vi "UHR-Fleezers Control (host) - 12.7c.vi"() -> ()   [LabVIEW 2012] (continued)
                  n359 = local read "Stop All"() -> (w575:bool)
                  n360 = Or(x=w577, y=w572) -> (x .or. y?=w574:bool)
                  n361 = Not(x=w574) -> (.not. x?=w576:bool)
                  n362 = Compound Arithmetic op=OR(w575, w576) -> (w573:bool)
                }
              }
              n363 = node-c288() -> ()  [unwired: 2 out]
            }
            n364 = node-c288(w409) -> ()  [unwired: 1 out]
          }
        }
      }
      event "Fl. Triggered...": Value Change {
        n365 = event-data() -> ()  [unwired: 7 out]
        n366 = case shown="True" "Fl. Triggered..." {
          frame False {
          }
          frame True {
            n367 = node-c288() -> (w588:T23)  [unwired: 4 out]
            n368 = timed-loop {
              timing: w588 -> [_]
              timing-out: [_] -> w587
              tunnel: "Action" -> [w596]
              shift-right: [w593] -> _
              shift-left: u8 255 -> [w595]
              shift-right: [w590] -> _
              shift-left: 255 -> [w592]
              stop <- w589 stop-if-true
              # "Reset confocal spot"
              n369 = node-c288() -> ()  [unwired: 2 out]
              n370 = flat-sequence {
                tunnel: w596 -> [w616]
                tunnel: w595 -> [w615]
                tunnel: [w614] -> w594
                tunnel: w592 -> [w601]
                tunnel: [w600] -> w591
                tunnel: [w995] -> w589
                tunnel: w594 -> [w994]
                tunnel: [w994] -> w593
                tunnel: [w993] -> w590
                tunnel: w591 -> [w993]
                frame #0 {
                  n371 = local read "Delta Fl. 2"() -> (w613:dbl)
                  n372 = local read "Delta Fl. 1"() -> (w608:dbl)
                  n373 = Multiply(x="Fl. Delta Thresh. (kHz)", y=1000.0) -> (x*y=w603:dbl)
                  n374 = Select(t=w608, s="APD to Watch", f=w613) -> (s? t:f=w604:dbl)
                  n375 = Greater?(x=w604, y=w603) -> (0:w609:bool)
                  n376 = Or(x="Force Yank", y=w609) -> (x .or. y?=w607:bool)
                  n377 = And(x=w607, y="Yank when?") -> (x .and. y?=w605:bool)
                  n378 = case shown="False" w605 {
                    tunnel: w616 -> [w619 w820]
                    tunnel: w615 -> [w621 w816]
                    tunnel: [w621 w814] -> w614
                    tunnel: w604 -> [w627 _]
                    tunnel: w603 -> [w626 _]
                    tunnel: "Force Yank" -> [w624 _]
                    tunnel: w601 -> [w623 w813]
                    tunnel: [w622 w813] -> w600
                    frame False {
                      n379 = Negate(x=w626) -> (-x=w618:dbl)
                      n380 = local write "Fl. High"(TRUE ("Fl. High")) -> ()
                      n381 = Less?(x=w627, y=w618) -> (x < y?=w625:bool)
                      n382 = Or(x=w624, y=w625) -> (x .or. y?=w620:bool)
                      n383 = case shown="True" w620 {
                        tunnel: w623 -> [w628 w638]
                        tunnel: [w628 w637] -> w622
                        tunnel: w619 -> [_ w636]
                        frame False {
                        }
                        frame True {
                          n384 = flat-sequence {
                            tunnel: w638 -> [w644]
                            tunnel: w636 -> [w641]
                            tunnel: [w643] -> w635
                            tunnel: [w642] -> w634
                            tunnel: [w641] -> w633
                            tunnel: w632 -> [w640]
                            tunnel: [w640] -> w631
                            tunnel: w630 -> [w639]
                            tunnel: [w639] -> w629
                            tunnel: [w715] -> w637
                            tunnel: w635 -> [w715]
                            tunnel: w634 -> [w714]
                            tunnel: w633 -> [w713]
                            tunnel: w631 -> [w712]
                            tunnel: w629 -> [w711]
                            frame #0 {
                              n385 = call <vilib>:"Beep.vi"() -> ()  [unwired: 12 in]
                              n386 = local write "Waiting"(FALSE ("Waiting")) -> ()
                              n387 = Increment(x=w644) -> (x+1=w643:i32)
                              n388 = case shown="\"Image\"" w641 {
                                tunnel: w643 -> [_ w649 _]
                                frame "Alarm", Default {
                                }
                                frame "Yank" {
                                n389 = flat-sequence {
                                tunnel: w649 -> [w652]
                                tunnel: [w651] -> w648
                                tunnel: [w650] -> w647
                                tunnel: w648 -> [w662]
                                tunnel: w647 -> [w663]
                                frame #0 {
                                n390 = local read "Yank Delay (s)"() -> (w655:dbl)
                                n391 = local read "N Array El"() -> (w650:u8)
                                n392 = Quotient & Remainder(x=w652, y=w650) -> (x-y*floor(x/y)=w651:i32)  [unwired: 1 out]
                                n393 = Multiply(x=w655, y=1000.0) -> (x*y=w653:dbl)
                                n394 = Wait (ms)(milliseconds to wait=w653) -> ()  [unwired: 1 out]
                                }
                                frame #1 {
                                n395 = local read "Yank to which?"() -> (w657:bool)
                                n396 = local read "Random Choice"() -> (w667:bool)
                                n397 = local read "Yank to Trap Delta (MHz)"() -> (w660:dbl[])
                                n398 = local read "Yank to SP"() -> (w661:dbl[])
                                n399 = Random Number (0-1)() -> (number: 0 to 1=w666:dbl)
                                n400 = Multiply(x=w663, y=w666) -> (x*y=w665:dbl)
                                n401 = Round Toward -Infinity(1:w665) -> (0:w664:dbl)
                                n402 = Select(t=w664, s=w667, f=w662) -> (s? t:f=w658:dbl)
                                n403 = Select(t=w660, s=w657, f=w661) -> (s? t:f=w659:dbl[])
                                n404 = Index Array(array=w659, index=w658) -> (element=w656:dbl)
                                n405 = case shown="True" w657 {
                                tunnel: w656 -> [w668 w695]
                                frame False {
                                n406 = flat-sequence {
                                tunnel: w668 -> [w669]
                                frame #0 {
                                n407 = property on="Trap Pos FB SP" class="DigNum (strict)"("Val(Sgnl)"=w669) -> ()  [unwired: 2 in, 2 out]
                                }
                                frame #1 {
                                n408 = Wait (ms)(milliseconds to wait=u32 700) -> ()  [unwired: 1 out]
                                }
                                frame #2 {
                                n409 = local read "Action (%)"() -> (w674:dbl)
                                n410 = Absolute Value(x=w674) -> (abs(x)=w673:dbl)
                                n411 = Greater?(x=w673, y=70.0) -> (0:w671:bool)
                                n412 = property on="Remove Action Offset" class="Bool (strict)"("Val(Sgnl)"=w671) -> ()  [unwired: 2 in, 2 out]
                                }
                                frame #3 {
                                n413 = for {
                                N: 4 -> [_]
                                n414 = flat-sequence {
                                frame #0 {
                                n415 = Wait (ms)(milliseconds to wait=u32 500) -> ()  [unwired: 1 out]
                                }
                                frame #1 {
                                n416 = local read "Action (%)"() -> (w680:dbl)
                                n417 = Absolute Value(x=w680) -> (abs(x)=w679:dbl)
                                n418 = Greater?(x=w679, y=70.0) -> (0:w677:bool)
                                n419 = property on="Remove Action Offset" class="Bool (strict)"("Val(Sgnl)"=w677) -> ()  [unwired: 2 in, 2 out]
                                }
                                }
                                }
                                }
                                frame #4 {
                                n420 = Wait (ms)(milliseconds to wait=u32 500) -> ()  [unwired: 1 out]
                                }
                                frame #5 {
                                n421 = local read "Mean"() -> (w688:dbl)
                                n422 = Greater?(x=w688, y=11.0) -> (0:w682:bool)
                                n423 = Not(x=w682) -> (.not. x?=w683:bool)
                                n424 = And(x=w683, y="Shift confocal") -> (x .and. y?=w685:bool)
                                n425 = And(x=w682, y="Shift confocal") -> (x .and. y?=w686:bool)
                                n426 = case shown="True" w686 {
                                frame False {
                                }
                                frame True {
                                n427 = local read "Confocal Y 2 (V)"() -> (w692:dbl)
                                n428 = local read "Confocal X 2 (V)"() -> (w691:dbl)
                                n429 = property on="AO1" class="Slide (strict)"("Val(Sgnl)"=w692) -> ()  [unwired: 2 in, 2 out]
                                n430 = property on="AO2" class="Slide (strict)"("Val(Sgnl)"=w691) -> ()  [unwired: 2 in, 2 out]
                                }
                                }
                                n431 = case shown="True" w685 {
                                frame False {
                                }
                                frame True {
                                n432 = local read "Confocal Y 1 (V)"() -> (w690:dbl)
                                n433 = local read "Confocal X 1 (V)"() -> (w689:dbl)
                                n434 = property on="AO1" class="Slide (strict)"("Val(Sgnl)"=w690) -> ()  [unwired: 2 in, 2 out]
                                n435 = property on="AO2" class="Slide (strict)"("Val(Sgnl)"=w689) -> ()  [unwired: 2 in, 2 out]
                                }
                                }
                                }
                                frame #6 {
                                n436 = Wait (ms)(milliseconds to wait=u32 1500) -> ()  [unwired: 1 out]
                                }
                                frame #7 {
                                n437 = property on="Rem fb disp offset" class="Bool (strict)"("Val(Sgnl)"=TRUE ("Value (Signaling)")) -> ()  [unwired: 2 in, 2 out]
                                }
                                }
                                }
                                frame True {
                                n438 = flat-sequence {
                                tunnel: w695 -> [w696]
                                frame #0 {
                                n439 = property on="Trap Delta (MHz)" class="DigNum (strict)"("Val(Sgnl)"=w696) -> ()  [unwired: 2 in, 2 out]
                                }
                                frame #1 {
                                n440 = Wait (ms)(milliseconds to wait=u32 500) -> ()  [unwired: 1 out]
                                }
                                frame #2 {
                                n441 = local read "Shift confocal"() -> (w702:bool)
                                n442 = local read "Mean"() -> (w704:dbl)
                                n443 = Greater?(x=w704, y=11.0) -> (0:w701:bool)
                                n444 = Not(x=w701) -> (.not. x?=w700:bool)
                                n445 = And(x=w700, y=w702) -> (x .and. y?=w698:bool)
                                n446 = And(x=w701, y=w702) -> (x .and. y?=w699:bool)
                                n447 = case shown="True" w699 {
                                frame False {
                                }
                                frame True {
                                n448 = local read "Confocal Y 2 (V)"() -> (w708:dbl)
                                n449 = local read "Confocal X 2 (V)"() -> (w707:dbl)
                                n450 = property on="AO2" class="Slide (strict)"("Val(Sgnl)"=w707) -> ()  [unwired: 2 in, 2 out]
                                n451 = property on="AO1" class="Slide (strict)"("Val(Sgnl)"=w708) -> ()  [unwired: 2 in, 2 out]
                                }
                                }
                                n452 = case shown="True" w698 {
                                frame False {
                                }
                                frame True {
                                n453 = local read "Confocal X 1 (V)"() -> (w705:dbl)
                                n454 = local read "Confocal Y 1 (V)"() -> (w706:dbl)
                                n455 = property on="AO2" class="Slide (strict)"("Val(Sgnl)"=w705) -> ()  [unwired: 2 in, 2 out]
                                n456 = property on="AO1" class="Slide (strict)"("Val(Sgnl)"=w706) -> ()  [unwired: 2 in, 2 out]
                                }
                                }
                                }
                                }
                                }
                                }
                                }
                                }
                                }
                                frame "Image" {
                                n457 = property on="Confocal Image" class="Bool (strict)"("Val(Sgnl)"=TRUE ("Value (Signaling)")) -> ()  [unwired: 2 in, 2 out]
                                }
                              }
                              n458 = local write "Fl. High"(FALSE ("Fl. High")) -> ()
                              n459 = local read "Time (s)"() -> (w642:dbl)
                            }
                            frame #1 {
                              n460 = case shown="True" "Auto F Reset" {
                                tunnel: w714 -> [_ w719]
                                tunnel: w713 -> [_ w718]
                                tunnel: w712 -> [_ w717]
                                tunnel: w711 -> [_ w716]
                                frame False {
                                }
                                frame True {
                                n461 = node-c288() -> (w721:T23)  [unwired: 4 in]
                                n462 = timed-loop {
                                timing: w721 -> [_]
                                timing-out: [_] -> w720
                                tunnel: w719 -> [w726]
                                tunnel: w718 -> [w725]
                                tunnel: w717 -> [w724]
                                tunnel: w716 -> [w723]
                                stop <- w722 stop-if-true
                                n463 = node-c288() -> ()  [unwired: 1 in, 1 out]
                                n464 = local read "Fl. Delta Thresh. (kHz)"() -> (w735:dbl)
                                n465 = local read "APD to Watch"() -> (w736:bool)
                                n466 = local read "Delta Fl. 1"() -> (w737:dbl)
                                n467 = local read "Delta Fl. 2"() -> (w738:dbl)
                                n468 = local read "Fl. Triggered..."() -> (w729:bool)
                                n469 = local read "Stop All"() -> (w730:bool)
                                n470 = local read "Reset Force"() -> (w728:bool)
                                n471 = Multiply(x=w735, y=1000.0) -> (x*y=w733:dbl)
                                n472 = Select(t=w737, s=w736, f=w738) -> (s? t:f=w732:dbl)
                                n473 = Not(x=w729) -> (.not. x?=w727:bool)
                                n474 = Greater?(x=w732, y=w733) -> (0:w731:bool)
                                n475 = Compound Arithmetic op=OR(w731, w730, w727, w728) -> (w722:bool)
                                n476 = case shown="True" w722 {
                                tunnel: w726 -> [_ w742]
                                tunnel: w725 -> [_ w746]
                                tunnel: w724 -> [_ w745]
                                tunnel: w723 -> [_ w744]
                                frame False {
                                }
                                frame True {
                                n477 = case shown="\"Yank\"" w746 {
                                tunnel: w745 -> [_ w756]
                                tunnel: w744 -> [_ w754]
                                frame "Image", Default {
                                }
                                frame "Yank" {
                                n478 = flat-sequence {
                                tunnel: [w759] -> w757
                                tunnel: w756 -> [w759]
                                tunnel: [w758] -> w755
                                tunnel: w754 -> [w758]
                                tunnel: w757 -> [w765]
                                tunnel: w755 -> [w763]
                                frame #0 {
                                n479 = local read "Yank Delay (s)"() -> (w762:dbl)
                                n480 = Multiply(x=w762, y=1000.0) -> (x*y=w760:dbl)
                                n481 = Wait (ms)(milliseconds to wait=w760) -> ()  [unwired: 1 out]
                                }
                                frame #1 {
                                n482 = local read "Yank to which?"() -> (w764:bool)
                                n483 = case shown="False" w764 {
                                tunnel: w765 -> [_ w793]
                                tunnel: w763 -> [w766 _]
                                frame False {
                                n484 = flat-sequence {
                                tunnel: w766 -> [w767]
                                frame #0 {
                                n485 = property on="Trap Pos FB SP" class="DigNum (strict)"("Val(Sgnl)"=w767) -> ()  [unwired: 2 in, 2 out]
                                }
                                frame #1 {
                                n486 = Wait (ms)(milliseconds to wait=u32 700) -> ()  [unwired: 1 out]
                                }
                                frame #2 {
                                n487 = local read "Action (%)"() -> (w772:dbl)
                                n488 = Absolute Value(x=w772) -> (abs(x)=w771:dbl)
                                n489 = Greater?(x=w771, y=70.0) -> (0:w769:bool)
                                n490 = property on="Remove Action Offset" class="Bool (strict)"("Val(Sgnl)"=w769) -> ()  [unwired: 2 in, 2 out]
                                }
                                frame #3 {
                                n491 = for {
                                N: 4 -> [_]
                                n492 = flat-sequence {
                                frame #0 {
                                n493 = Wait (ms)(milliseconds to wait=u32 500) -> ()  [unwired: 1 out]
                                }
                                frame #1 {
                                n494 = local read "Action (%)"() -> (w778:dbl)
                                n495 = Absolute Value(x=w778) -> (abs(x)=w777:dbl)
                                n496 = Greater?(x=w777, y=70.0) -> (0:w775:bool)
                                n497 = property on="Remove Action Offset" class="Bool (strict)"("Val(Sgnl)"=w775) -> ()  [unwired: 2 in, 2 out]
                                }
                                }
                                }
                                }
                                frame #4 {
                                n498 = Wait (ms)(milliseconds to wait=u32 500) -> ()  [unwired: 1 out]
                                }
                                frame #5 {
                                n499 = local read "Shift confocal"() -> (w783:bool)
                                n500 = local read "Mean"() -> (w786:dbl)
                                n501 = Greater?(x=w786, y=11.0) -> (0:w782:bool)
                                n502 = Not(x=w782) -> (.not. x?=w781:bool)
                                n503 = And(x=w782, y=w783) -> (x .and. y?=w784:bool)
                                n504 = And(x=w781, y=w783) -> (x .and. y?=w780:bool)
                                n505 = case shown="True" w784 {
                                frame False {
                                }
                                frame True {
                                n506 = local read "Confocal X 2 (V)"() -> (w789:dbl)
                                n507 = local read "Confocal Y 2 (V)"() -> (w790:dbl)
                                n508 = property on="AO2" class="Slide (strict)"("Val(Sgnl)"=w789) -> ()  [unwired: 2 in, 2 out]
                                n509 = property on="AO1" class="Slide (strict)"("Val(Sgnl)"=w790) -> ()  [unwired: 2 in, 2 out]
                                }
                                }
                                n510 = case shown="True" w780 {
                                frame False {
                                }
                                frame True {
                                n511 = local read "Confocal Y 1 (V)"() -> (w788:dbl)
                                n512 = local read "Confocal X 1 (V)"() -> (w787:dbl)
                                n513 = property on="AO1" class="Slide (strict)"("Val(Sgnl)"=w788) -> ()  [unwired: 2 in, 2 out]
                                n514 = property on="AO2" class="Slide (strict)"("Val(Sgnl)"=w787) -> ()  [unwired: 2 in, 2 out]
                                }
                                }
                                }
                                frame #6 {
                                n515 = Wait (ms)(milliseconds to wait=u32 1500) -> ()  [unwired: 1 out]
                                }
                                frame #7 {
                                n516 = property on="Rem fb disp offset" class="Bool (strict)"("Val(Sgnl)"=TRUE ("Value (Signaling)")) -> ()  [unwired: 2 in, 2 out]
                                }
                                }
                                }
                                frame True {
                                n517 = flat-sequence {
                                tunnel: w793 -> [w794]
                                frame #0 {
                                n518 = property on="Trap Delta (MHz)" class="DigNum (strict)"("Val(Sgnl)"=w794) -> ()  [unwired: 2 in, 2 out]
                                }
                                frame #1 {
                                n519 = Wait (ms)(milliseconds to wait=u32 500) -> ()  [unwired: 1 out]
                                }
                                frame #2 {
                                n520 = local read "Shift confocal"() -> (w800:bool)
                                n521 = local read "Mean"() -> (w801:dbl)
                                n522 = Greater?(x=w801, y=11.0) -> (0:w799:bool)
                                n523 = And(x=w799, y=w800) -> (x .and. y?=w797:bool)
                                n524 = Not(x=w799) -> (.not. x?=w798:bool)
                                n525 = And(x=w798, y=w800) -> (x .and. y?=w796:bool)
                                n526 = case shown="True" w797 {
                                frame False {
                                }
                                frame True {
                                n527 = local read "Confocal Y 2 (V)"() -> (w806:dbl)
                                n528 = local read "Confocal X 2 (V)"() -> (w805:dbl)
                                n529 = property on="AO1" class="Slide (strict)"("Val(Sgnl)"=w806) -> ()  [unwired: 2 in, 2 out]
                                n530 = property on="AO2" class="Slide (strict)"("Val(Sgnl)"=w805) -> ()  [unwired: 2 in, 2 out]
                                }
                                }
                                n531 = case shown="True" w796 {
                                frame False {
                                }
                                frame True {
                                n532 = local read "Confocal Y 1 (V)"() -> (w804:dbl)
                                n533 = local read "Confocal X 1 (V)"() -> (w803:dbl)
                                n534 = property on="AO2" class="Slide (strict)"("Val(Sgnl)"=w803) -> ()  [unwired: 2 in, 2 out]
                                n535 = property on="AO1" class="Slide (strict)"("Val(Sgnl)"=w804) -> ()  [unwired: 2 in, 2 out]
                                }
                                }
                                }
                                }
                                }
                                }
                                }
                                }
                                }
                                }
                                n536 = local read "Time (s)"() -> (w741:dbl)
                                n537 = Subtract(x=w742, y=w741) -> (x-y=w753:dbl)
                                n538 = Number To Decimal String(number=w753, width (-)=i16 0) -> (decimal integer string=w751:string)
                                n539 = Concatenate Strings(w751, " s fluorescence event") -> (w748:string)
                                n540 = local read "Messages"() -> (w749:string)
                                n541 = local write "Duration (s)"(w753) -> ()
                                n542 = call "Update messages.vi"("Message to add"=w748, "Old message string"=w749) -> ("New message string"=w747:string)
                                n543 = local write "Messages"(w747) -> ()
                                n544 = call <vilib>:"Beep.vi"() -> ()  [unwired: 12 in]
                                n545 = local write "Reset Force"(FALSE ("Force Reset")) -> ()
                                n546 = local write "Fl. High"(TRUE ("Fl. High")) -> ()
                                n547 = local write "Waiting"(TRUE ("Waiting")) -> ()
                                }
                                }
                                n548 = node-c288() -> ()  [unwired: 1 in, 1 out]
                                }
                                n549 = node-c288(w720) -> ()  [unwired: 1 out]
                                }
                              }
                            }
                          }
                          n550 = local read "Trap Delta (MHz)"() -> (w632:dbl)
                          n551 = local read "Trap Pos FB SP"() -> (w630:fxp<+/-,16,1>)
                        }
                      }
                    }
                    frame True {
                      n552 = flat-sequence {
                        tunnel: w817 -> [w827]
                        tunnel: [w827] -> w821
                        tunnel: w820 -> [w826]
                        tunnel: [w826] -> w819
                        tunnel: [w825] -> w818
                        tunnel: w816 -> [w824]
                        tunnel: [w823] -> w815
                        tunnel: w812 -> [w822]
                        tunnel: [w822] -> w811
                        tunnel: w821 -> [w897]
                        tunnel: w819 -> [w896]
                        tunnel: w818 -> [w895]
                        tunnel: w815 -> [w894]
                        tunnel: w811 -> [w893]
                        tunnel: [w894] -> w814
                        frame #0 {
                          n553 = call <vilib>:"Beep.vi"() -> ()  [unwired: 3 in, 9 out]
                          n554 = local write "Waiting"(FALSE ("Waiting")) -> ()
                          n555 = Increment(x=w824) -> (x+1=w823:u8)
                          n556 = case shown="\"Yank\"" w826 {
                            tunnel: w823 -> [_ _ w833]
                            frame "Image" {
                              n557 = property on="Confocal Image" class="Bool (strict)"("Val(Sgnl)"=TRUE ("Value (Signaling)")) -> ()  [unwired: 2 in, 2 out]
                            }
                            frame "Alarm", Default {
                            }
                            frame "Yank" {
                              n558 = flat-sequence {
                                tunnel: w833 -> [w836]
                                tunnel: [w835] -> w832
                                tunnel: ["N Array El"] -> w831
                                tunnel: w832 -> [w850]
                                tunnel: w831 -> [w846]
                                frame #0 {
                                n559 = Multiply(x="Yank Delay (s)", y=1000.0) -> (x*y=w839:dbl)
                                n560 = Quotient & Remainder(x=w836, y="N Array El") -> (x-y*floor(x/y)=w835:u8)  [unwired: 1 out]
                                n561 = Wait (ms)(milliseconds to wait=w839) -> ()  [unwired: 1 out]
                                }
                                frame #1 {
                                n562 = Random Number (0-1)() -> (number: 0 to 1=w847:dbl)
                                n563 = Multiply(x=w846, y=w847) -> (x*y=w845:dbl)
                                n564 = Round Toward -Infinity(1:w845) -> (0:w844:dbl)
                                n565 = Select(t=w844, s="Random Choice", f=w850) -> (s? t:f=w848:dbl)
                                n566 = Select(t="Yank to Trap Delta (MHz)", s="Yank to which?", f="Yank to SP") -> (s? t:f=w841:dbl[])
                                n567 = Index Array(array=w841, index=w848) -> (element=w851:dbl)
                                n568 = case shown="False" "Yank to which?" {
                                tunnel: w851 -> [w852 w878]
                                frame False {
                                n569 = flat-sequence {
                                tunnel: w852 -> [w853]
                                frame #0 {
                                n570 = property on="Trap Pos FB SP" class="DigNum (strict)"("Val(Sgnl)"=w853) -> ()  [unwired: 2 in, 2 out]
                                }
                                frame #1 {
                                n571 = Wait (ms)(milliseconds to wait=u32 700) -> ()  [unwired: 1 out]
                                }
                                frame #2 {
                                n572 = local read "Action (%)"() -> (w858:dbl)
                                n573 = Absolute Value(x=w858) -> (abs(x)=w857:dbl)
                                n574 = Greater?(x=w857, y=70.0) -> (0:w855:bool)
                                n575 = property on="Remove Action Offset" class="Bool (strict)"("Val(Sgnl)"=w855) -> ()  [unwired: 2 in, 2 out]
                                }
                                frame #3 {
                                n576 = for {
                                N: 4 -> [_]
                                n577 = flat-sequence {
                                frame #0 {
                                n578 = Wait (ms)(milliseconds to wait=u32 500) -> ()  [unwired: 1 out]
                                }
                                frame #1 {
                                n579 = local read "Action (%)"() -> (w864:dbl)
                                n580 = Absolute Value(x=w864) -> (abs(x)=w863:dbl)
                                n581 = Greater?(x=w863, y=70.0) -> (0:w861:bool)
                                n582 = property on="Remove Action Offset" class="Bool (strict)"("Val(Sgnl)"=w861) -> ()  [unwired: 2 in, 2 out]
                                }
                                }
                                }
                                }
                                frame #4 {
                                n583 = local read "Shift confocal"() -> (w868:bool)
                                n584 = local read "Mean"() -> (w871:dbl)
                                n585 = Greater?(x=w871, y=11.0) -> (0:w867:bool)
                                n586 = Not(x=w867) -> (.not. x?=w866:bool)
                                n587 = And(x=w866, y=w868) -> (x .and. y?=w865:bool)
                                n588 = And(x=w867, y=w868) -> (x .and. y?=w869:bool)
                                n589 = case shown="True" w869 {
                                frame False {
                                }
                                frame True {
                                n590 = local read "Confocal X 2 (V)"() -> (w874:dbl)
                                n591 = local read "Confocal Y 2 (V)"() -> (w875:dbl)
                                n592 = property on="AO2" class="Slide (strict)"("Val(Sgnl)"=w874) -> ()  [unwired: 2 in, 2 out]
                                n593 = property on="AO1" class="Slide (strict)"("Val(Sgnl)"=w875) -> ()  [unwired: 2 in, 2 out]
                                }
                                }
                                n594 = case shown="True" w865 {
                                frame False {
                                }
                                frame True {
                                n595 = local read "Confocal X 1 (V)"() -> (w872:dbl)
                                n596 = local read "Confocal Y 1 (V)"() -> (w873:dbl)
                                n597 = property on="AO1" class="Slide (strict)"("Val(Sgnl)"=w873) -> ()  [unwired: 2 in, 2 out]
                                n598 = property on="AO2" class="Slide (strict)"("Val(Sgnl)"=w872) -> ()  [unwired: 2 in, 2 out]
                                }
                                }
                                }
                                frame #5 {
                                n599 = Wait (ms)(milliseconds to wait=u32 1500) -> ()  [unwired: 1 out]
                                }
                                frame #6 {
                                n600 = property on="Rem fb disp offset" class="Bool (strict)"("Val(Sgnl)"=TRUE ("Value (Signaling)")) -> ()  [unwired: 2 in, 2 out]
                                }
                                }
                                }
                                frame True {
                                n601 = flat-sequence {
                                tunnel: w878 -> [w879]
                                frame #0 {
                                n602 = property on="Trap Delta (MHz)" class="DigNum (strict)"("Val(Sgnl)"=w879) -> ()  [unwired: 2 in, 2 out]
                                }
                                frame #1 {
                                n603 = Wait (ms)(milliseconds to wait=u32 500) -> ()  [unwired: 1 out]
                                }
                                frame #2 {
                                n604 = local read "Shift confocal"() -> (w883:bool)
                                n605 = local read "Mean"() -> (w881:dbl)
                                n606 = Greater?(x=w881, y=11.0) -> (0:w884:bool)
                                n607 = Not(x=w884) -> (.not. x?=w885:bool)
                                n608 = And(x=w885, y=w883) -> (x .and. y?=w887:bool)
                                n609 = And(x=w884, y=w883) -> (x .and. y?=w886:bool)
                                n610 = case shown="True" w886 {
                                frame False {
                                }
                                frame True {
                                n611 = local read "Confocal Y 2 (V)"() -> (w891:dbl)
                                n612 = local read "Confocal X 2 (V)"() -> (w890:dbl)
                                n613 = property on="AO1" class="Slide (strict)"("Val(Sgnl)"=w891) -> ()  [unwired: 2 in, 2 out]
                                n614 = property on="AO2" class="Slide (strict)"("Val(Sgnl)"=w890) -> ()  [unwired: 2 in, 2 out]
                                }
                                }
                                n615 = case shown="True" w887 {
                                frame False {
                                }
                                frame True {
                                n616 = local read "Confocal X 1 (V)"() -> (w888:dbl)
                                n617 = local read "Confocal Y 1 (V)"() -> (w889:dbl)
                                n618 = property on="AO2" class="Slide (strict)"("Val(Sgnl)"=w888) -> ()  [unwired: 2 in, 2 out]
                                n619 = property on="AO1" class="Slide (strict)"("Val(Sgnl)"=w889) -> ()  [unwired: 2 in, 2 out]
                                }
                                }
                                }
                                }
                                }
                                }
                                }
                              }
                            }
                          }
                          n620 = local read "Time (s)"() -> (w825:dbl)
                          "Fl. High" <- TRUE ("Yanking")
                        }
                        frame #1 {
                          n621 = local read "Auto F Reset"() -> (w892:bool)
                          n622 = case shown="True" w892 {
                            tunnel: w897 -> [_ w901]
                            tunnel: w896 -> [_ w900]
                            tunnel: w895 -> [_ w899]
                            tunnel: w893 -> [_ w898]
                            frame False {
                            }
                            frame True {
                              n623 = node-c288() -> (w903:T23)  [unwired: 4 out]
                              n624 = timed-loop {
                                timing: w903 -> [_]
                                timing-out: [_] -> w902
                                tunnel: w901 -> [w921]
                                tunnel: w900 -> [w920]
                                tunnel: w899 -> [w919]
                                tunnel: w898 -> [w918]
                                stop <- w904 stop-if-true
                                n625 = node-c288() -> ()  [unwired: 2 out]
                                n626 = local read "Fl. Delta Thresh. (kHz)"() -> (w912:dbl)
                                n627 = local read "Fl. Triggered..."() -> (w917:bool)
                                n628 = local read "Delta Fl. 1"() -> (w908:dbl)
                                n629 = local read "Delta Fl. 2"() -> (w906:dbl)
                                n630 = local read "Stop All"() -> (w915:bool)
                                n631 = local read "APD to Watch"() -> (w907:bool)
                                n632 = Select(t=w908, s=w907, f=w906) -> (s? t:f=w905:dbl)
                                n633 = Not(x=w917) -> (.not. x?=w916:bool)
                                n634 = Multiply(x=w912, y=1000.0) -> (x*y=w911:dbl)
                                n635 = Negate(x=w911) -> (-x=w910:dbl)
                                n636 = Less?(x=w905, y=w910) -> (x < y?=w914:bool)
                                n637 = Compound Arithmetic op=OR(w914, w915, w916, "Reset Force") -> (w904:bool)
                                n638 = case shown="True" w904 {
                                tunnel: w921 -> [_ w936]
                                tunnel: w920 -> [_ w935]
                                tunnel: w919 -> [_ w925]
                                tunnel: w918 -> [_ w927]
                                frame False {
                                }
                                frame True {
                                n639 = local read "Time (s)"() -> (w926:dbl)
                                n640 = case shown="\"Yank\"" w935 {
                                tunnel: w936 -> [_ w939]
                                tunnel: w927 -> [_ w937]
                                frame "Image", Default {
                                }
                                frame "Yank" {
                                n641 = flat-sequence {
                                tunnel: [w945] -> w940
                                tunnel: w939 -> [w945]
                                tunnel: [w941] -> w938
                                tunnel: w937 -> [w941]
                                tunnel: w940 -> [w948]
                                tunnel: w938 -> [w946]
                                frame #0 {
                                n642 = local read "Yank Delay (s)"() -> (w944:dbl)
                                n643 = Multiply(x=w944, y=1000.0) -> (x*y=w942:dbl)
                                n644 = Wait (ms)(milliseconds to wait=w942) -> ()  [unwired: 1 out]
                                }
                                frame #1 {
                                n645 = local read "Yank to which?"() -> (w947:bool)
                                n646 = case shown="False" w947 {
                                tunnel: w948 -> [_ w975]
                                tunnel: w946 -> [w949 _]
                                frame False {
                                n647 = flat-sequence {
                                tunnel: w949 -> [w950]
                                frame #0 {
                                n648 = property on="Trap Pos FB SP" class="DigNum (strict)"("Val(Sgnl)"=w950) -> ()  [unwired: 2 in, 2 out]
                                }
                                frame #1 {
                                n649 = Wait (ms)(milliseconds to wait=u32 700) -> ()  [unwired: 1 out]
                                }
                                frame #2 {
                                n650 = local read "Action (%)"() -> (w955:dbl)
                                n651 = Absolute Value(x=w955) -> (abs(x)=w954:dbl)
                                n652 = Greater?(x=w954, y=70.0) -> (0:w952:bool)
                                n653 = property on="Remove Action Offset" class="Bool (strict)"("Val(Sgnl)"=w952) -> ()  [unwired: 2 in, 2 out]
                                }
                                frame #3 {
                                n654 = for {
                                N: 4 -> [_]
                                n655 = flat-sequence {
                                frame #0 {
                                n656 = Wait (ms)(milliseconds to wait=u32 500) -> ()  [unwired: 1 out]
                                }
                                frame #1 {
                                n657 = local read "Action (%)"() -> (w961:dbl)
                                n658 = Absolute Value(x=w961) -> (abs(x)=w960:dbl)
                                n659 = Greater?(x=w960, y=70.0) -> (0:w958:bool)
                                n660 = property on="Remove Action Offset" class="Bool (strict)"("Val(Sgnl)"=w958) -> ()  [unwired: 2 in, 2 out]
                                }
                                }
                                }
                                }
                                frame #4 {
                                n661 = local read "Shift confocal"() -> (w966:bool)
                                n662 = local read "Mean"() -> (w968:dbl)
                                n663 = Greater?(x=w968, y=11.0) -> (0:w965:bool)
                                n664 = Not(x=w965) -> (.not. x?=w964:bool)
                                n665 = And(x=w965, y=w966) -> (x .and. y?=w963:bool)
                                n666 = And(x=w964, y=w966) -> (x .and. y?=w962:bool)
                                n667 = case shown="True" w963 {
                                frame False {
                                }
                                frame True {
                                n668 = local read "Confocal Y 2 (V)"() -> (w972:dbl)
                                n669 = local read "Confocal X 2 (V)"() -> (w971:dbl)
                                n670 = property on="AO2" class="Slide (strict)"("Val(Sgnl)"=w971) -> ()  [unwired: 2 in, 2 out]
                                n671 = property on="AO1" class="Slide (strict)"("Val(Sgnl)"=w972) -> ()  [unwired: 2 in, 2 out]
                                }
                                }
                                n672 = case shown="True" w962 {
                                frame False {
                                }
                                frame True {
                                n673 = local read "Confocal X 1 (V)"() -> (w969:dbl)
                                n674 = local read "Confocal Y 1 (V)"() -> (w970:dbl)
                                n675 = property on="AO1" class="Slide (strict)"("Val(Sgnl)"=w970) -> ()  [unwired: 2 in, 2 out]
                                n676 = property on="AO2" class="Slide (strict)"("Val(Sgnl)"=w969) -> ()  [unwired: 2 in, 2 out]
                                }
                                }
                                }
                                frame #5 {
                                n677 = Wait (ms)(milliseconds to wait=u32 1500) -> ()  [unwired: 1 out]
                                }
                                frame #6 {
                                n678 = property on="Rem fb disp offset" class="Bool (strict)"("Val(Sgnl)"=TRUE ("Value (Signaling)")) -> ()  [unwired: 2 in, 2 out]
                                }
                                }
                                }
                                frame True {
                                n679 = flat-sequence {
                                tunnel: w975 -> [w976]
                                frame #0 {
                                n680 = property on="Trap Delta (MHz)" class="DigNum (strict)"("Val(Sgnl)"=w976) -> ()  [unwired: 2 in, 2 out]
                                }
                                frame #1 {
                                n681 = Wait (ms)(milliseconds to wait=u32 500) -> ()  [unwired: 1 out]
                                }
                                frame #2 {
                                n682 = local read "Shift confocal"() -> (w982:bool)
                                n683 = local read "Mean"() -> (w984:dbl)
                                n684 = Greater?(x=w984, y=11.0) -> (0:w981:bool)
                                n685 = Not(x=w981) -> (.not. x?=w980:bool)
                                n686 = And(x=w981, y=w982) -> (x .and. y?=w979:bool)
                                n687 = And(x=w980, y=w982) -> (x .and. y?=w978:bool)
                                n688 = case shown="True" w979 {
                                frame False {
                                }
                                frame True {
                                n689 = local read "Confocal Y 2 (V)"() -> (w988:dbl)
                                n690 = local read "Confocal X 2 (V)"() -> (w987:dbl)
                                n691 = property on="AO2" class="Slide (strict)"("Val(Sgnl)"=w987) -> ()  [unwired: 2 in, 2 out]
                                n692 = property on="AO1" class="Slide (strict)"("Val(Sgnl)"=w988) -> ()  [unwired: 2 in, 2 out]
                                }
                                }
                                n693 = case shown="True" w978 {
                                frame False {
                                }
                                frame True {
                                n694 = local read "Confocal Y 1 (V)"() -> (w986:dbl)
                                n695 = local read "Confocal X 1 (V)"() -> (w985:dbl)
                                n696 = property on="AO2" class="Slide (strict)"("Val(Sgnl)"=w985) -> ()  [unwired: 2 in, 2 out]
                                n697 = property on="AO1" class="Slide (strict)"("Val(Sgnl)"=w986) -> ()  [unwired: 2 in, 2 out]
                                }
                                }
                                }
                                }
                                }
                                }
                                }
                                }
                                }
                                }
                                n698 = local read "Messages"() -> (w934:string)
                                n699 = Subtract(x=w926, y=w925) -> (x-y=w932:dbl)
                                "Duration (s)" <- w932
                                n700 = Number To Decimal String(number=w932, width (-)=i16 0) -> (decimal integer string=w930:string)
                                n701 = Concatenate Strings(w930, " s fluorescence event." ("string")) -> (w928:string)
                                n702 = call "Update messages.vi"("Message to add"=w928, "Old message string"=w934) -> ("New message string"=w933:string)
                                n703 = local write "Reset Force"(FALSE ("Reset Force")) -> ()
                                n704 = local write "Waiting"(TRUE ("Waiting")) -> ()
                                n705 = local write "Messages"(w933) -> ()
                                n706 = local write "Fl. High"(FALSE ("Fl. High")) -> ()
                                n707 = call <vilib>:"Beep.vi"() -> ()  [unwired: 3 in, 9 out]
                                }
                                }
                                n708 = node-c288() -> ()  [unwired: 2 out]
                              }
                              n709 = node-c288(w902) -> ()  [unwired: 1 out]
                            }
                          }
                        }
                      }
                      n710 = local read "Trap Delta (MHz)"() -> (w817:dbl)
                      n711 = local read "Trap Pos FB SP"() -> (w812:fxp<+/-,16,1>)
                    }
                  }
                }
                frame #1 {
                  n712 = local read "Stop All"() -> (w998:bool)
                  n713 = local read "Fl. Triggered..."() -> (w996:bool)
                  n714 = Not(x=w996) -> (.not. x?=w997:bool)
                  n715 = Or(x=w997, y=w998) -> (x .or. y?=w995:bool)
                }
              }
              n716 = case shown="True" w589 {
                frame False {
                }
                frame True {
                  n717 = local read "Confocal Y 1 (V)"() -> (w599:dbl)
                  n718 = local read "Confocal X 1 (V)"() -> (w598:dbl)
                  n719 = property on="AO2" class="Slide (strict)"("Val(Sgnl)"=w598) -> ()  [unwired: 2 in, 2 out]
                  n720 = property on="AO1" class="Slide (strict)"("Val(Sgnl)"=w599) -> ()  [unwired: 2 in, 2 out]
                }
              }
              n721 = case shown="True" w589 {
                frame False {
                }
                frame True {
                  w597 = FALSE ("Fl. High")
                  n722 = local write "Waiting"(w597) -> ()
                  n723 = local write "Fl. High"(w597) -> ()
                }
              }
              n724 = node-c288() -> ()  [unwired: 2 out]
            }
            n725 = node-c288(w587) -> ()  [unwired: 1 out]
          }
        }
      }
      event "Stop All": Value Change {
        n726 = event-data() -> ()  [unwired: 7 out]
        n727 = local read "Stop All"() -> (w1003:bool)
      }
    }
    n728 = node-c288() -> ()  [unwired: 2 out]
  }
  n729 = timed-loop "Basic control parameters (all FPGA settings, other basic controls)" {
    tunnel: w1 -> [w1012]
    shift-right: [w1011] -> _
    shift-left: errorcluster {"status"=FALSE, "code"=0, "source"=""} ("error out") -> [w1010]
    tunnel: [w1009] -> _
    timing: w133 -> [_]
    timing-out: [_] -> w132
    tunnel: w106 -> [w1008]
    tunnel: w78 -> [w1007]
    tunnel: w77 -> [w1006]
    tunnel: w76 -> [w1005]
    tunnel: w75 -> [w1004]
    stop <- w1009 stop-if-true
    n730 = node-c288() -> ()  [unwired: 2 out]
    n731 = event shown="[6] \"BD 1 Frequency 1 (MHz)\", \"BD 1 Frequency 2 (MHz)\", \"BD 1 Frequency 3 (MHz)\", \"BD 2 Frequency 1 (MHz)\", \"BD 2 Frequency 2 (MHz)\", \"BD 2 Frequency 3 (MHz)\", \"Trap Delta (MHz)\", \"Update all trap values\": Value Change" {
      selector: _ -> [_ _ _ _ _ _ _ _ _ _ _ _ _ _ _ _ _ _ _ _ _ _ _ _ _ _ _ _ _ _ _ _ _ _ _ _ _ _ _ _ _ _ _ _ _ _ _ _ _ _ _ _ _ _ _ _ _ _ _ _ _ _ _ _ _ _ _ _ _ _ _ _ _ _]
      dyn-events: _ -> [_ _ _ _ _ _ _ _ _ _ _ _ _ _ _ _ _ _ _ _ _ _ _ _ _ _ _ _ _ _ _ _ _ _ _ _ _ _ _ _ _ _ _ _ _ _ _ _ _ _ _ _ _ _ _ _ _ _ _ _ _ _ _ _ _ _ _ _ _ _ _ _ _ _]
      timeout: _ -> [_ _ _ _ _ _ _ _ _ _ _ _ _ _ _ _ _ _ _ _ _ _ _ _ _ _ _ _ _ _ _ _ _ _ _ _ _ _ _ _ _ _ _ _ _ _ _ _ _ _ _ _ _ _ _ _ _ _ _ _ _ _ _ _ _ _ _ _ _ _ _ _ _ _]
      tunnel: w1012 -> [w1053 _ _ _ w1091 _ w1114 _ _ _ _ w1180 _ _ w1230 w1236 w1243 w1248 w1321 _ w1337 w1362 w1383 w1404 w1424 w1453 w1479 w1482 w1486 w1581 w1586 w1624 _ w1659 w1663 w1674 w1678 w1682 _ w1690 _ _ _ _ _ _ _ _ _ _ _ _ _ _ _ _ _ w2068 _ w2085 _ w2092 w2110 _ w2117 w2125 w2140 w2156 w2162 _ w2171 _ w2190 _]